vi "3kButtonsSys36x36.vi"() -> ()   [LabVIEW 2011] (continued)
  in  "folder_bell":bool
  in  "folder_add":bool
  in  "folder":bool
  in  "fog":bool
  in  "flower":bool
  in  "flood_it":bool
  in  "flickr":bool
  in  "flex_builder":bool
  in  "flex":bool
  in  "flask_empty":bool
  in  "flask":bool
  in  "flashlight_shine":bool
  in  "flashlight":bool
  in  "flashdisk":bool
  in  "flamingo":bool
  in  "flag_zimbabwe":bool
  in  "flag_zambia":bool
  in  "flag_yemen":bool
  in  "flag_yellow":bool
  in  "flag_wwf":bool
  in  "flag_wto":bool
  in  "flag_wallis_and_futuna":bool
  in  "flag_wales":bool
  in  "flag_virgin_islands":bool
  in  "flag_vietnam":bool
  in  "flag_venezuela":bool
  in  "flag_vatican_city":bool
  in  "flag_vanuatu":bool
  in  "flag_uzbekistan":bool
  in  "flag_usa":bool
  in  "flag_uruquay":bool
  in  "flag_united_nations":bool
  in  "flag_united_arab_emirates":bool
  in  "flag_unesco":bool
  in  "flag_ukraine":bool
  in  "flag_uganda":bool
  in  "flag_tuvalu":bool
  in  "flag_turks_and_caicos_islands":bool
  in  "flag_turkmenistan":bool
  in  "flag_turkey":bool
  in  "flag_tunisia":bool
  in  "flag_trinidad_and_tobago":bool
  in  "flag_tonga":bool
  in  "flag_togo":bool
  in  "flag_tibet":bool
  in  "flag_thailand":bool
  in  "flag_tanzania":bool
  in  "flag_tajikistan":bool
  in  "flag_taiwan":bool
  in  "flag_syria":bool
  in  "flag_switzerland":bool
  in  "flag_sweden":bool
  in  "flag_swaziland":bool
  in  "flag_suriname":bool
  in  "flag_sudan":bool
  in  "flag_sri_lanka":bool
  in  "flag_spain":bool
  in  "flag_south_korea":bool
  in  "flag_south_georgia":bool
  in  "flag_south_africa":bool
  in  "flag_somalia":bool
  in  "flag_solomon_islands":bool
  in  "flag_slovenia":bool
  in  "flag_slovakia":bool
  in  "flag_singapore":bool
  in  "flag_sierra_leone":bool
  in  "flag_seychelles":bool
  in  "flag_serbia_montenegro":bool
  in  "flag_senegal":bool
  in  "flag_scotland":bool
  in  "flag_saudi_arabia":bool
  in  "flag_sao_tome_and_principe":bool
  in  "flag_san_marino":bool
  in  "flag_samoa":bool
  in  "flag_saint_vincent_and_grenadines":bool
  in  "flag_saint_pierre_and_miquelon":bool
  in  "flag_saint_lucia":bool
  in  "flag_saint_kitts_and_nevis":bool
  in  "flag_saint_helena":bool
  in  "flag_rwanda":bool
  in  "flag_russia":bool
  in  "flag_romania":bool
  in  "flag_red_cross":bool
  in  "flag_red":bool
  in  "flag_qatar":bool
  in  "flag_purple":bool
  in  "flag_puerto_rico":bool
  in  "flag_portugal":bool
  in  "flag_poland":bool
  in  "flag_pitcairn_islands":bool
  in  "flag_pink":bool
  in  "flag_philippines":bool
  in  "flag_peru":bool
  in  "flag_paraquay":bool
  in  "flag_papua_new_guinea":bool
  in  "flag_panama":bool
  in  "flag_palau":bool
  in  "flag_pakistan":bool
  in  "flag_orange":bool
  in  "flag_oman":bool
  in  "flag_olympic":bool
  in  "flag_norway":bool
  in  "flag_northern_mariana_islands":bool
  in  "flag_north_korea":bool
  in  "flag_norfolk_islands":bool
  in  "flag_niue":bool
  in  "flag_nigeria":bool
  in  "flag_niger":bool
  in  "flag_nicaragua":bool
  in  "flag_new_zealand":bool
  in  "flag_new":bool
  in  "flag_netherlands_antilles":bool
  in  "flag_netherlands":bool
  in  "flag_nepal":bool
  in  "flag_nauru":bool
  in  "flag_nato":bool
  in  "flag_namibia":bool
  in  "flag_mozambique":bool
  in  "flag_morocco":bool
  in  "flag_montserrat":bool
  in  "flag_mongolia":bool
  in  "flag_monaco":bool
  in  "flag_moldova":bool
  in  "flag_micronesia":bool
  in  "flag_mexico":bool
  in  "flag_mauritius":bool
  in  "flag_mauretania":bool
  in  "flag_martinique":bool
  in  "flag_marshall_islands":bool
  in  "flag_malta":bool
  in  "flag_mali":bool
  in  "flag_maledives":bool
  in  "flag_malaysia":bool
  in  "flag_malawi":bool
  in  "flag_madagascar":bool
  in  "flag_macedonia":bool
  in  "flag_macau":bool
  in  "flag_luxembourg":bool
  in  "flag_lithuania":bool
  in  "flag_liechtenstein":bool
  in  "flag_libya":bool
  in  "flag_liberia":bool
  in  "flag_lesotho":bool
  in  "flag_lebanon":bool
  in  "flag_latvia":bool
  in  "flag_laos":bool
  in  "flag_kyrgyzstan":bool
  in  "flag_kuwait":bool
  in  "flag_kiribati":bool
  in  "flag_kenya":bool
  in  "flag_kazakhstan":bool
  in  "flag_jordan":bool
  in  "flag_jersey":bool
  in  "flag_japan":bool
  in  "flag_jamaica":bool
  in  "flag_italy":bool
  in  "flag_israel":bool
  in  "flag_isle_of_man":bool
  in  "flag_ireland":bool
  in  "flag_iraq":bool
  in  "flag_iran":bool
  in  "flag_indonesia":bool
  in  "flag_india":bool
  in  "flag_iceland":bool
  in  "flag_hungary":bool
  in  "flag_hot":bool
  in  "flag_hong_kong":bool
  in  "flag_honduras":bool
  in  "flag_haiti":bool
  in  "flag_guyana":bool
  in  "flag_guinea_bissau":bool
  in  "flag_guinea":bool
  in  "flag_guernsey":bool
  in  "flag_guatemala":bool
  in  "flag_guam":bool
  in  "flag_grenada":bool
  in  "flag_greenland":bool
  in  "flag_green":bool
  in  "flag_greece":bool
  in  "flag_great_britain":bool
  in  "flag_gibraltar":bool
  in  "flag_ghana":bool
  in  "flag_germany":bool
  in  "flag_georgia":bool
  in  "flag_gambia":bool
  in  "flag_gabon":bool
  in  "flag_french_polynesia":bool
  in  "flag_france":bool
  in  "flag_finland":bool
  in  "flag_finish":bool
  in  "flag_fiji":bool
  in  "flag_faroe_islands":bool
  in  "flag_falkland_islands":bool
  in  "flag_european_union":bool
  in  "flag_ethiopia":bool
  in  "flag_estonia":bool
  in  "flag_eritrea":bool
  in  "flag_equatorial_guinea":bool
  in  "flag_equador":bool
  in  "flag_england":bool
  in  "flag_el_salvador":bool
  in  "flag_egypt":bool
  in  "flag_east_timor":bool
  in  "flag_dominican_republic":bool
  in  "flag_dominica":bool
  in  "flag_djibouti":bool
  in  "flag_denmark":bool
  in  "flag_czech_republic":bool
  in  "flag_cyprus":bool
  in  "flag_cuba":bool
  in  "flag_croatia":bool
  in  "flag_cote_divoire":bool
  in  "flag_costa_rica":bool
  in  "flag_cope_verde":bool
  in  "flag_cook_islands":bool
  in  "flag_congo_republic":bool
  in  "flag_congo_democratic_republic":bool
  in  "flag_comoros":bool
  in  "flag_colombia":bool
  in  "flag_china":bool
  in  "flag_chile":bool
  in  "flag_chad":bool
  in  "flag_central_african_republic":bool
  in  "flag_cayman_islands":bool
  in  "flag_canada":bool
  in  "flag_cameroon":bool
  in  "flag_cambodia":bool
  in  "flag_burundi":bool
  in  "flag_burma":bool
  in  "flag_burkina_faso":bool
  in  "flag_bulgaria":bool
  in  "flag_brunei":bool
  in  "flag_british_virgin_islands":bool
  in  "flag_british_indian_ocean":bool
  in  "flag_brazil":bool
  in  "flag_boy_scout":bool
  in  "flag_botswana":bool
  in  "flag_bosnia":bool
  in  "flag_bolivia":bool
  in  "flag_blue":bool
  in  "flag_bhutan":bool
  in  "flag_bermuda":bool
  in  "flag_benin":bool
  in  "flag_belize":bool
  in  "flag_belgium":bool
  in  "flag_belarus":bool
  in  "flag_barbados":bool
  in  "flag_bangladesh":bool
  in  "flag_bahrain":bool
  in  "flag_bahamas":bool
  in  "flag_azerbaijan":bool
  in  "flag_austria":bool
  in  "flag_australia":bool
  in  "flag_aruba":bool
  in  "flag_armenia":bool
  in  "flag_argentina":bool
  in  "flag_antigua_and_barbuda":bool
  in  "flag_anguilla":bool
  in  "flag_angola":bool
  in  "flag_andorra":bool
  in  "flag_american_samoa":bool
  in  "flag_algeria":bool
  in  "flag_albania":bool
  in  "flag_airfield_vehicle_safety":bool
  in  "flag_afghanistan":bool
  in  "flag_3":bool
  in  "flag_2":bool
  in  "flag_1":bool
  in  "fishfinder":bool
  in  "firewall_burn":bool
  in  "firewall":bool
  in  "firefox":bool
  in  "fire_extinguisher":bool
  in  "fire_damage":bool
  in  "fire":bool
  in  "fingerprint":bool
  in  "find":bool
  in  "finance":bool
  in  "filter_delete":bool
  in  "filter_add":bool
  in  "filter":bool
  in  "film_save":bool
  in  "film_photo":bool
  in  "film_link":bool
  in  "film_key":bool
  in  "film_go":bool
  in  "film_error":bool
  in  "film_edit":bool
  in  "film_delete":bool
  in  "film_add":bool
  in  "film":bool
  in  "fill":bool
  in  "file_manager":bool
  in  "file_extension_zip":bool
  in  "file_extension_xpi":bool
  in  "file_extension_xls":bool
  in  "file_extension_wps":bool
  in  "file_extension_wmv":bool
  in  "file_extension_wma":bool
  in  "file_extension_wav":bool
  in  "file_extension_vob":bool
  in  "file_extension_vcd":bool
  in  "file_extension_txt":bool
  in  "file_extension_ttf":bool
  in  "file_extension_torrent":bool
  in  "file_extension_tmp":bool
  in  "file_extension_tif":bool
  in  "file_extension_thm":bool
  in  "file_extension_tgz":bool
  in  "file_extension_swf":bool
  in  "file_extension_ss":bool
  in  "file_extension_sitx":bool
  in  "file_extension_sit":bool
  in  "file_extension_ses":bool
  in  "file_extension_sea":bool
  in  "file_extension_rtf":bool
  in  "file_extension_rmvb":bool
  in  "file_extension_rm":bool
  in  "file_extension_rar":bool
  in  "file_extension_ram":bool
  in  "file_extension_qxd":bool
  in  "file_extension_qbw":bool
  in  "file_extension_qbb":bool
  in  "file_extension_pub":bool
  in  "file_extension_ptb":bool
  in  "file_extension_pst":bool
  in  "file_extension_psd":bool
  in  "file_extension_ps":bool
  in  "file_extension_pps":bool
  in  "file_extension_png":bool
  in  "file_extension_pdf":bool
  in  "file_extension_ogg":bool
  in  "file_extension_mswmm":bool
  in  "file_extension_msi":bool
  in  "file_extension_mpg":bool
  in  "file_extension_mpeg":bool
  in  "file_extension_mp4":bool
  in  "file_extension_mp2":bool
  in  "file_extension_mov":bool
  in  "file_extension_mid":bool
  in  "file_extension_mdb":bool
  in  "file_extension_mcd":bool
  in  "file_extension_m4v":bool
  in  "file_extension_m4p":bool
  in  "file_extension_m4b":bool
  in  "file_extension_m4a":bool
  in  "file_extension_log":bool
  in  "file_extension_lnk":bool
  in  "file_extension_jpg":bool
  in  "file_extension_jpeg":bool
  in  "file_extension_jar":bool
  in  "file_extension_iso":bool
  in  "file_extension_indd":bool
  in  "file_extension_ifo":bool
  in  "file_extension_html":bool
  in  "file_extension_htm":bool
  in  "file_extension_hqx":bool
  in  "file_extension_gz":bool
  in  "file_extension_gif":bool
  in  "file_extension_flv":bool
  in  "file_extension_fla":bool
  in  "file_extension_exe":bool
  in  "file_extension_eps":bool
  in  "file_extension_eml":bool
  in  "file_extension_dwg":bool
  in  "file_extension_dvf":bool
  in  "file_extension_dss":bool
  in  "file_extension_doc":bool
  in  "file_extension_dmg":bool
  in  "file_extension_dll":bool
  in  "file_extension_divx":bool
  in  "file_extension_dat":bool
  in  "file_extension_chm":bool
  in  "file_extension_cdr":bool
  in  "file_extension_cdl":bool
  in  "file_extension_cda":bool
  in  "file_extension_cbr":bool
  in  "file_extension_cab":bool
  in  "file_extension_bup":bool
  in  "file_extension_bmp":bool
  in  "file_extension_bin":bool
  in  "file_extension_bat":bool
  in  "file_extension_asx":bool
  in  "file_extension_asf":bool
  in  "file_extension_amr":bool
  in  "file_extension_aiff":bool
  in  "file_extension_aif":bool
  in  "file_extension_ai":bool
  in  "file_extension_ace":bool
  in  "file_extension_7z":bool
  in  "file_extension_3gp":bool
  in  "female":bool
  in  "feed_magnify":bool
  in  "feed_key":bool
  in  "feed_go":bool
  in  "feed_error":bool
  in  "feed_edit":bool
  in  "feed_disk":bool
  in  "feed_delete":bool
  in  "feed_add":bool
  in  "feed":bool
  in  "fedora":bool
  in  "fax":bool
  in  "fatcow":bool
  in  "factory":bool
  in  "facebook":bool
  in  "faberge_egg":bool
  in  "eye_red":bool
  in  "eye_close":bool
  in  "eye":bool
  in  "extract_foreground_objects":bool
  in  "external":bool
  in  "export_excel":bool
  in  "exclamation":bool
  in  "evernote":bool
  in  "events":bool
  in  "evacuator":bool
  in  "escimo_pie":bool
  in  "error_go":bool
  in  "error_delete":bool
  in  "error_add":bool
  in  "error":bool
  in  "envelope_string":bool
  in  "envelope":bool
  in  "entity":bool
  in  "emotion_zedz":bool
  in  "emotion_wink":bool
  in  "emotion_whist":bool
  in  "emotion_what":bool
  in  "emotion_waii":bool
  in  "emotion_waaaht":bool
  in  "emotion_vampire":bool
  in  "emotion_unshaven":bool
  in  "emotion_unhappy":bool
  in  "emotion_too_sad":bool
  in  "emotion_tongue":bool
  in  "emotion_tire":bool
  in  "emotion_terminator":bool
  in  "emotion_sweat":bool
  in  "emotion_surrender":bool
  in  "emotion_sure":bool
  in  "emotion_suprised":bool
  in  "emotion_stupid":bool
  in  "emotion_star":bool
  in  "emotion_spy":bool
  in  "emotion_spiderman":bool
  in  "emotion_smile":bool
  in  "emotion_sleep":bool
  in  "emotion_skull":bool
  in  "emotion_silent":bool
  in  "emotion_sick":bool
  in  "emotion_shocked":bool
  in  "emotion_shame":bool
  in  "emotion_sad":bool
  in  "emotion_red":bool
  in  "emotion_rap":bool
  in  "emotion_question":bool
  in  "emotion_pumpkin":bool
  in  "emotion_pirate":bool
  in  "emotion_nosebleed":bool
  in  "emotion_ninja":bool
  in  "emotion_nerd":bool
  in  "emotion_mummy":bool
  in  "emotion_money":bool
  in  "emotion_misdoubt":bool
  in  "emotion_medic":bool
  in  "emotion_matrix":bool
  in  "emotion_mad":bool
  in  "emotion_love":bool
  in  "emotion_kissed":bool
  in  "emotion_kiss":bool
  in  "emotion_jason":bool
  in  "emotion_japan":bool
  in  "emotion_hypnotized":bool
  in  "emotion_hungry":bool
  in  "emotion_horror":bool
  in  "emotion_hitler":bool
  in  "emotion_happy":bool
  in  "emotion_hand_flower":bool
  in  "emotion_haha":bool
  in  "emotion_grin":bool
  in  "emotion_greedy":bool
  in  "emotion_go":bool
  in  "emotion_girl":bool
  in  "emotion_ghost":bool
  in  "emotion_gear":bool
  in  "emotion_franken":bool
  in  "emotion_flower_dead":bool
  in  "emotion_fan":bool
  in  "emotion_face_panda":bool
  in  "emotion_face_monkey":bool
  in  "emotion_eyes_droped":bool
  in  "emotion_exciting":bool
  in  "emotion_evolution":bool
  in  "emotion_evilgrin":bool
  in  "emotion_dribble":bool
  in  "emotion_doubt":bool
  in  "emotion_diver":bool
  in  "emotion_devil":bool
  in  "emotion_dead":bool
  in  "emotion_david_blaine":bool
  in  "emotion_darth_wader":bool
  in  "emotion_cyclops":bool
  in  "emotion_cry":bool
  in  "emotion_crazy_rabbit":bool
  in  "emotion_crazy":bool
  in  "emotion_cool":bool
  in  "emotion_confuse":bool
  in  "emotion_confident":bool
  in  "emotion_cold":bool
  in  "emotion_clown":bool
  in  "emotion_bye_bye":bool
  in  "emotion_bubblegum":bool
  in  "emotion_bloody":bool
  in  "emotion_bigsmile":bool
  in  "emotion_beaten":bool
  in  "emotion_beat_brick":bool
  in  "emotion_batman":bool
  in  "emotion_baffle":bool
  in  "emotion_bad_smelly":bool
  in  "emotion_bad_egg":bool
  in  "emotion_baby":bool
  in  "emotion_angry":bool
  in  "emotion_anger":bool
  in  "emotion_angel":bool
  in  "emotion_amazing":bool
  in  "emotion_alien":bool
  in  "emotion_ah":bool
  in  "emotion_after_boom":bool
  in  "emotion_adore":bool
  in  "ember":bool
  in  "emails_stack":bool
  in  "emails":bool
  in  "email_to_friend":bool
  in  "email_send_receive":bool
  in  "email_open_image":bool
  in  "email_open":bool
  in  "email_link":bool
  in  "email_go":bool
  in  "email_forward":bool
  in  "email_error":bool
  in  "email_edit":bool
  in  "email_delete":bool
  in  "email_attach":bool
  in  "email_at_sign":bool
  in  "email_air":bool
  in  "email_add":bool
  in  "email":bool
  in  "elements":bool
  in  "electric_guitar":bool
  in  "ehow":bool
  in  "egyptian_pyramid":bool
  in  "education":bool
  in  "edit_path":bool
  in  "edit_mathematics":bool
  in  "edit_free":bool
  in  "edit_diff":bool
  in  "edit_chain":bool
  in  "echeck":bool
  in  "ebay":bool
  in  "earth_night":bool
  in  "ear_listen":bool
  in  "e_book_reader_white":bool
  in  "e_book_reader_black":bool
  in  "dynamite":bool
  in  "dvd_link":bool
  in  "dvd_key":bool
  in  "dvd_go":bool
  in  "dvd_error":bool
  in  "dvd_edit":bool
  in  "dvd_delete":bool
  in  "dvd_add":bool
  in  "dvd":bool
  in  "drum":bool
  in  "drugs_com":bool
  in  "drop":bool
  in  "drive_web":bool
  in  "drive_user":bool
  in  "drive_rename":bool
  in  "drive_network":bool
  in  "drive_magnify":bool
  in  "drive_link":bool
  in  "drive_key":bool
  in  "drive_go":bool
  in  "drive_error":bool
  in  "drive_edit":bool
  in  "drive_disk":bool
  in  "drive_delete":bool
  in  "drive_cd_empty":bool
  in  "drive_cd":bool
  in  "drive_burn":bool
  in  "drive_add":bool
  in  "drive":bool
  in  "drink_empty":bool
  in  "drink":bool
  in  "drill":bool
  in  "dribbble":bool
  in  "drawer_open":bool
  in  "drawer":bool
  in  "draw_wave":bool
  in  "draw_vertex":bool
  in  "draw_star":bool
  in  "draw_spiral":bool
  in  "draw_smudge":bool
  in  "draw_ring":bool
  in  "draw_polyline":bool
  in  "draw_polygon_curves":bool
  in  "draw_polygon":bool
  in  "draw_points":bool
  in  "draw_path":bool
  in  "draw_line":bool
  in  "draw_island":bool
  in  "draw_ink":bool
  in  "draw_eraser":bool
  in  "draw_ellipse":bool
  in  "draw_dodge_burn":bool
  in  "draw_convolve":bool
  in  "draw_clone":bool
  in  "draw_calligraphic":bool
  in  "draw_airbrush":bool
  in  "download_for_windows":bool
  in  "download_for_mac":bool
  in  "download_for_linux":bool
  in  "download_cloud":bool
  in  "download":bool
  in  "down_jacket":bool
  in  "dopplr":bool
  in  "door_out":bool
  in  "door_open":bool
  in  "door_in":bool
  in  "door":bool
  in  "donut":bool
  in  "domain_template":bool
  in  "domain_names_advanced":bool
  in  "domain_name_monetization":bool
  in  "domain_name_investment":bool
  in  "domain_legal_issues":bool
  in  "domain_controversies":bool
  in  "domain_buying_selling":bool
  in  "dog":bool
  in  "documents_email":bool
  in  "document_yellow":bool
  in  "document_white_torn":bool
  in  "document_view_book":bool
  in  "document_vertical":bool
  in  "document_valid":bool
  in  "document_tree":bool
  in  "document_torn":bool
  in  "document_todo":bool
  in  "document_tag":bool
  in  "document_stand":bool
  in  "document_split":bool
  in  "document_spacing":bool
  in  "document_signature":bool
  in  "document_shred":bool
  in  "document_shapes":bool
  in  "document_rename":bool
  in  "document_redirect":bool
  in  "document_red":bool
  in  "document_quote":bool
  in  "document_properties":bool
  in  "document_prepare":bool
  in  "document_plus":bool
  in  "document_page_previous":bool
  in  "document_page_next":bool
  in  "document_page_last":bool
  in  "document_page":bool
  in  "document_num":bool
  in  "document_notes":bool
  in  "document_next":bool
  in  "document_move":bool
  in  "document_mark_as_final":bool
  in  "document_margins":bool
  in  "document_layout":bool
  in  "document_inspector":bool
  in  "document_inspect":bool
  in  "document_insert":bool
  in  "document_info":bool
  in  "document_index":bool
  in  "document_import":bool
  in  "document_image_ver":bool
  in  "document_image_hor":bool
  in  "document_image":bool
  in  "document_green":bool
  in  "document_font_wizard":bool
  in  "document_font":bool
  in  "document_export":bool
  in  "document_empty":bool
  in  "document_editing":bool
  in  "document_copies":bool
  in  "document_comments":bool
  in  "document_comment_below":bool
  in  "document_comment_behind":bool
  in  "document_comment_above":bool
  in  "document_check_compatibility":bool
  in  "document_center":bool
  in  "document_break":bool
  in  "document_black":bool
  in  "document_background":bool
  in  "document_back":bool
  in  "do_not_disturb":bool
  in  "dns_setting":bool
  in  "dns":bool
  in  "distribution_partnerships":bool
  in  "disk_multiple":bool
  in  "disk":bool
  in  "dish":bool
  in  "discover":bool
  in  "disconnect":bool
  in  "directory_listing":bool
  in  "direction":bool
  in  "dinersclub":bool
  in  "digital_signature_pen":bool
  in  "digital_signature":bool
  in  "digg":bool
  in  "dice":bool
  in  "diamond":bool
  in  "dialog":bool
  in  "diagramm":bool
  in  "diagnostic_chart":bool
  in  "devianart":bool
  in  "desktop":bool
  in  "designmoo":bool
  in  "design_float":bool
  in  "derivatives":bool
  in  "delicious":bool
  in  "delete":bool
  in  "decimal_more":bool
  in  "decimal_less":bool
  in  "debian":bool
  in  "ddr_memory":bool
  in  "date_task":bool
  in  "date_relation":bool
  in  "date_previous_gray":bool
  in  "date_previous":bool
  in  "date_next_gray":bool
  in  "date_next":bool
  in  "date_magnify":bool
  in  "date_link":bool
  in  "date_go":bool
  in  "date_error":bool
  in  "date_edit":bool
  in  "date_delete":bool
  in  "date_add":bool
  in  "date":bool
  in  "database_yellow":bool
  in  "database_table":bool
  in  "database_server":bool
  in  "database_save":bool
  in  "database_refresh":bool
  in  "database_red":bool
  in  "database_link":bool
  in  "database_lightning":bool
  in  "database_key":bool
  in  "database_green":bool
  in  "database_go":bool
  in  "database_gear":bool
  in  "database_error":bool
  in  "database_edit":bool
  in  "database_delete":bool
  in  "database_connect":bool
  in  "database_blue":bool
  in  "database_black":bool
  in  "database_add":bool
  in  "database":bool
  in  "data_table":bool
  in  "data_sort":bool
  in  "data_grid":bool
  in  "data_field":bool
  in  "data_chooser":bool
  in  "dashboard":bool
  in  "cutter":bool
  in  "cutlery":bool
  in  "cutleries":bool
  in  "cut_red":bool
  in  "cut":bool
  in  "cushion":bool
  in  "curtain":bool
  in  "cursor":bool
  in  "curriculum_vitae":bool
  in  "cup_silver":bool
  in  "cup_link":bool
  in  "cup_key":bool
  in  "cup_gold":bool
  in  "cup_go":bool
  in  "cup_error":bool
  in  "cup_edit":bool
  in  "cup_delete":bool
  in  "cup_bronze":bool
  in  "cup_add":bool
  in  "cup":bool
  in  "css_valid":bool
  in  "css_go":bool
  in  "css_delete":bool
  in  "css_add":bool
  in  "css_3":bool
  in  "css":bool
  in  "cruise_ship":bool
  in  "crown_silver":bool
  in  "crown_gold":bool
  in  "crown_bronze":bool
  in  "cross_shield":bool
  in  "cross_promotion_selling":bool
  in  "cross":bool
  in  "cricket":bool
  in  "creditcards":bool
  in  "credit":bool
  in  "creative_commons":bool
  in  "counter":bool
  in  "copyleft":bool
  in  "copying_and_distribution":bool
  in  "cooler":bool
  in  "cookies":bool
  in  "cookie_chocolate":bool
  in  "convert_gray_to_color":bool
  in  "convert_color_to_gray":bool
  in  "conversion_of_currency":bool
  in  "controller_error":bool
  in  "controller_delete":bool
  in  "controller_add":bool
  in  "controller":bool
  in  "controlbar":bool
  in  "control_stop_blue":bool
  in  "control_stop":bool
  in  "control_start_blue":bool
  in  "control_start":bool
  in  "control_rewind_blue":bool
  in  "control_rewind":bool
  in  "control_repeat_blue":bool
  in  "control_repeat":bool
  in  "control_power_blue":bool
  in  "control_power":bool
  in  "control_play_blue":bool
  in  "control_play":bool
  in  "control_pause_record":bool
  in  "control_pause_blue":bool
  in  "control_pause":bool
  in  "control_panel_branding":bool
  in  "control_panel_access":bool
  in  "control_panel":bool
  in  "control_fastforward_blue":bool
  in  "control_fastforward":bool
  in  "control_equalizer_blue":bool
  in  "control_equalizer":bool
  in  "control_end_blue":bool
  in  "control_end":bool
  in  "control_eject_blue":bool
  in  "control_eject":bool
  in  "control_cursor_blue":bool
  in  "control_cursor":bool
  in  "contrast_low":bool
  in  "contrast_increase":bool
  in  "contrast_high":bool
  in  "contrast_decrease":bool
  in  "contrast":bool
  in  "contact_email":bool
  in  "construction":bool
  in  "connect":bool
  in  "computer_link":bool
  in  "computer_key":bool
  in  "computer_go":bool
  in  "computer_error":bool
  in  "computer_edit":bool
  in  "computer_delete":bool
  in  "computer_add":bool
  in  "computer":bool
  in  "compress":bool
  in  "compile_warning":bool
  in  "compile_error":bool
  in  "compile":bool
  in  "compass":bool
  in  "company_generosity":bool
  in  "comments_twitter":bool
  in  "comments_facebook":bool
  in  "comments_delete":bool
  in  "comments_add":bool
  in  "comments":bool
  in  "comment_white":bool
  in  "comment_twitter_retwit":bool
  in  "comment_twitter_box":bool
  in  "comment_twitter":bool
  in  "comment_google":bool
  in  "comment_facebook_box":bool
  in  "comment_facebook":bool
  in  "comment_edit":bool
  in  "comment_delete":bool
  in  "comment_box":bool
  in  "comment_add":bool
  in  "comment":bool
  in  "combo_box":bool
  in  "columnchart":bool
  in  "column_two":bool
  in  "column_tree":bool
  in  "column_single":bool
  in  "column_right":bool
  in  "column_one":bool
  in  "column_left":bool
  in  "column_four":bool
  in  "column_double":bool
  in  "color_wheel":bool
  in  "color_swatches":bool
  in  "color_swatch":bool
  in  "color_picker_alternative":bool
  in  "color_picker":bool
  in  "color_management":bool
  in  "color_gradient":bool
  in  "color_adjustment_red":bool
  in  "color_adjustment_green":bool
  in  "color_adjustment_blue":bool
  in  "color_adjustment":bool
  in  "cold":bool
  in  "coins_in_hand":bool
  in  "coins_delete":bool
  in  "coins_add":bool
  in  "coins":bool
  in  "coin_stack_gold":bool
  in  "coin_single_silver":bool
  in  "coin_single_gold":bool
  in  "coin_single_cooper":bool
  in  "cog_go":bool
  in  "cog_error":bool
  in  "cog_edit":bool
  in  "cog_delete":bool
  in  "cog_add":bool
  in  "cog":bool
  in  "code":bool
  in  "cocacola":bool
  in  "co2":bool
  in  "clown_fish":bool
  in  "clock_stop":bool
  in  "clock_select_remain":bool
  in  "clock_red":bool
  in  "clock_play":bool
  in  "clock_pause":bool
  in  "clock_moon_phase":bool
  in  "clock_link":bool
  in  "clock_history_frame":bool
  in  "clock_go":bool
  in  "clock_error":bool
  in  "clock_edit":bool
  in  "clock_delete":bool
  in  "clock_add":bool
  in  "clock_45":bool
  in  "clock_15":bool
  in  "clock_":bool
  in  "clipboard_sign_out":bool
  in  "clipboard_sign":bool
  in  "clipboard_invoice":bool
  in  "clipboard_empty":bool
  in  "clip_splitter":bool
  in  "client_account_template":bool
  in  "cirrus":bool
  in  "circus":bool
  in  "cinema_ticket":bool
  in  "cigarette":bool
  in  "church":bool
  in  "christmas_tree":bool
  in  "chocolate_bite":bool
  in  "chocolate":bool
  in  "chinese_noodles":bool
  in  "children_cap":bool
  in  "chiken_leg":bool
  in  "chess_tower":bool
  in  "chess_horse":bool
  in  "cheque":bool
  in  "chefs_hat":bool
  in  "cheese":bool
  in  "checkerboard":bool
  in  "check_box":bool
  in  "chartplotter":bool
  in  "chart_up_color":bool
  in  "chart_stock":bool
  in  "chart_pie_link":bool
  in  "chart_pie_error":bool
  in  "chart_pie_edit":bool
  in  "chart_pie_delete":bool
  in  "chart_pie_alternative":bool
  in  "chart_pie_add":bool
  in  "chart_pie":bool
  in  "chart_organisation_delete":bool
  in  "chart_organisation_add":bool
  in  "chart_organisation":bool
  in  "chart_line_link":bool
  in  "chart_line_error":bool
  in  "chart_line_edit":bool
  in  "chart_line_delete":bool
  in  "chart_line_add":bool
  in  "chart_line":bool
  in  "chart_down_color":bool
  in  "chart_curve_link":bool
  in  "chart_curve_go":bool
  in  "chart_curve_error":bool
  in  "chart_curve_edit":bool
  in  "chart_curve_delete":bool
  in  "chart_curve_add":bool
  in  "chart_curve":bool
  in  "chart_column_2":bool
  in  "chart_column":bool
  in  "chart_bullseye":bool
  in  "chart_bar_link":bool
  in  "chart_bar_error":bool
  in  "chart_bar_edit":bool
  in  "chart_bar_delete":bool
  in  "chart_bar_add":bool
  in  "chart_bar":bool
  in  "change_password":bool
  in  "chameleon":bool
  in  "chair":bool
  in  "ceo":bool
  in  "centroid":bool
  in  "centos":bool
  in  "celsius":bool
  in  "cd_go":bool
  in  "cd_eject":bool
  in  "cd_edit":bool
  in  "cd_delete":bool
  in  "cd_case_empty":bool
  in  "cd_case":bool
  in  "cd_burn":bool
  in  "cd_add":bool
  in  "cd":bool
  in  "cctv_camera":bool
  in  "caution_radiation":bool
  in  "caution_high_voltage":bool
  in  "caution_board":bool
  in  "caution_biohazard":bool
  in  "cats_display":bool
  in  "caterpillar":bool
  in  "category_item_select":bool
  in  "category_item":bool
  in  "category_group_select":bool
  in  "category_group":bool
  in  "category":bool
  in  "categories":bool
  in  "cat":bool
  in  "cash_terminal":bool
  in  "cash_stack":bool
  in  "cash_register_2":bool
  in  "cash_register":bool
  in  "cart_remove":bool
  in  "cart_put":bool
  in  "cart_go":bool
  in  "cart_full":bool
  in  "cart_error":bool
  in  "cart_edit":bool
  in  "cart_delete":bool
  in  "cart_add":bool
  in  "cart":bool
  in  "cargo":bool
  in  "cards_binds":bool
  in  "cards_bind_address":bool
  in  "cards":bool
  in  "card_solo":bool
  in  "card_save":bool
  in  "card_sapphire":bool
  in  "card_money":bool
  in  "card_miles":bool
  in  "card_ipod":bool
  in  "card_import":bool
  in  "card_gold":bool
  in  "card_gift_2":bool
  in  "card_gift":bool
  in  "card_front":bool
  in  "card_export":bool
  in  "card_echeck":bool
  in  "card_discover_novus":bool
  in  "card_discover_black":bool
  in  "card_debit":bool
  in  "card_credit":bool
  in  "card_chip_silver":bool
  in  "card_chip_gold":bool
  in  "card_chase":bool
  in  "card_bank":bool
  in  "card_back":bool
  in  "card_apple":bool
  in  "card_amex_green":bool
  in  "card_amex_gray":bool
  in  "card_amex_gold":bool
  in  "card_amazon":bool
  in  "car_taxi":bool
  in  "car_delete":bool
  in  "car_add":bool
  in  "car":bool
  in  "cap":bool
  in  "canvas_size":bool
  in  "canvas":bool
  in  "candy_cane":bool
  in  "candlestickchart":bool
  in  "candle_2":bool
  in  "candle":bool
  in  "cancel":bool
  in  "camera_small":bool
  in  "camera_link":bool
  in  "camera_lens":bool
  in  "camera_go":bool
  in  "camera_error":bool
  in  "camera_edit":bool
  in  "camera_delete":bool
  in  "camera_black":bool
  in  "camera_add":bool
  in  "camera":bool
  in  "camcorder":bool
  in  "calendar_view_week":bool
  in  "calendar_view_month":bool
  in  "calendar_view_day":bool
  in  "calendar_link":bool
  in  "calendar_edit":bool
  in  "calendar_delete":bool
  in  "calendar_copy":bool
  in  "calendar_add":bool
  in  "calendar":bool
  in  "calculator_link":bool
  in  "calculator_error":bool
  in  "calculator_edit":bool
  in  "calculator_delete":bool
  in  "calculator_black":bool
  in  "calculator_add":bool
  in  "calculator":bool
  in  "cake":bool
  in  "cactus":bool
  in  "buzz":bool
  in  "buttonbar":bool
  in  "button":bool
  in  "butterfly":bool
  in  "bus":bool
  in  "burro":bool
  in  "bullet_yellow":bool
  in  "bullet_wrench":bool
  in  "bullet_world":bool
  in  "bullet_word":bool
  in  "bullet_white":bool
  in  "bullet_vector":bool
  in  "bullet_valid":bool
  in  "bullet_user":bool
  in  "bullet_up":bool
  in  "bullet_toggle_plus":bool
  in  "bullet_toggle_minus":bool
  in  "bullet_textfield":bool
  in  "bullet_table":bool
  in  "bullet_star":bool
  in  "bullet_red":bool
  in  "bullet_purple":bool
  in  "bullet_powerpoint":bool
  in  "bullet_pink":bool
  in  "bullet_picture":bool
  in  "bullet_php":bool
  in  "bullet_palette":bool
  in  "bullet_orange":bool
  in  "bullet_office":bool
  in  "bullet_medal":bool
  in  "bullet_magnify":bool
  in  "bullet_link":bool
  in  "bullet_lightning":bool
  in  "bullet_key":bool
  in  "bullet_green":bool
  in  "bullet_go":bool
  in  "bullet_gear":bool
  in  "bullet_flash":bool
  in  "bullet_find":bool
  in  "bullet_feed":bool
  in  "bullet_excel":bool
  in  "bullet_error":bool
  in  "bullet_edit":bool
  in  "bullet_dvd":bool
  in  "bullet_down":bool
  in  "bullet_document":bool
  in  "bullet_disk":bool
  in  "bullet_delete":bool
  in  "bullet_database":bool
  in  "bullet_connect":bool
  in  "bullet_code_red":bool
  in  "bullet_code":bool
  in  "bullet_chart":bool
  in  "bullet_cd":bool
  in  "bullet_camera":bool
  in  "bullet_burn":bool
  in  "bullet_bulb_on":bool
  in  "bullet_bulb_off":bool
  in  "bullet_bug":bool
  in  "bullet_brush":bool
  in  "bullet_blue":bool
  in  "bullet_black":bool
  in  "bullet_bell":bool
  in  "bullet_back":bool
  in  "bullet_attach":bool
  in  "bullet_arrow_up":bool
  in  "bullet_arrow_top":bool
  in  "bullet_arrow_right_2":bool
  in  "bullet_arrow_right":bool
  in  "bullet_arrow_left_2":bool
  in  "bullet_arrow_left":bool
  in  "bullet_arrow_down":bool
  in  "bullet_arrow_bottom":bool
  in  "bullet_archive":bool
  in  "bullet_add":bool
  in  "bulb":bool
  in  "building_link":bool
  in  "building_key":bool
  in  "building_go":bool
  in  "building_error":bool
  in  "building_edit":bool
  in  "building_delete":bool
  in  "building_add":bool
  in  "building":bool
  in  "bug_link":bool
  in  "bug_go":bool
  in  "bug_error":bool
  in  "bug_edit":bool
  in  "bug_delete":bool
  in  "bug_add":bool
  in  "bug":bool
  in  "bucket_truck":bool
  in  "bubblechart":bool
  in  "brushes":bool
  in  "broom":bool
  in  "brightkite":bool
  in  "briefcase":bool
  in  "bricks":bool
  in  "brick_link":bool
  in  "brick_go":bool
  in  "brick_error":bool
  in  "brick_edit":bool
  in  "brick_delete":bool
  in  "brick_add":bool
  in  "brick":bool
  in  "breeze":bool
  in  "bread":bool
  in  "brain_trainer":bool
  in  "brain":bool
  in  "boxing_glove":bool
  in  "box_search":bool
  in  "box_open":bool
  in  "box_front":bool
  in  "box_down":bool
  in  "box_closed":bool
  in  "box":bool
  in  "bow":bool
  in  "border_color":bool
  in  "border_2_top":bool
  in  "border_2_right":bool
  in  "border_2_outer":bool
  in  "border_2_left":bool
  in  "border_2_bottom":bool
  in  "border_1d_top":bool
  in  "border_1d_right":bool
  in  "border_1d_left":bool
  in  "border_1d_bottom":bool
  in  "border_1d_around":bool
  in  "border_1_ver":bool
  in  "border_1_top":bool
  in  "border_1_right":bool
  in  "border_1_outer":bool
  in  "border_1_none":bool
  in  "border_1_middle":bool
  in  "border_1_left":bool
  in  "border_1_hor":bool
  in  "border_1_bottom":bool
  in  "border_1":bool
  in  "boomerang":bool
  in  "bookshelf":bool
  in  "books_stack":bool
  in  "books":bool
  in  "bookmark_red":bool
  in  "bookmark":bool
  in  "book_spelling":bool
  in  "book_previous":bool
  in  "book_picture":bool
  in  "book_open":bool
  in  "book_next":bool
  in  "book_link":bool
  in  "book_key":bool
  in  "book_keeping":bool
  in  "book_go":bool
  in  "book_error":bool
  in  "book_edit":bool
  in  "book_delete":bool
  in  "book_addresses":bool
  in  "book_add":bool
  in  "book":bool
  in  "bomb":bool
  in  "board_game":bool
  in  "bluetooth":bool
  in  "blueprints":bool
  in  "blueprint_horizontal":bool
  in  "blueprint":bool
  in  "blogs":bool
  in  "blogger":bool
  in  "blackboard_sum":bool
  in  "blackboard_steps":bool
  in  "blackboard_empty":bool
  in  "blackboard_drawing":bool
  in  "blackberry_white":bool
  in  "blackberry_messenger":bool
  in  "blackberry":bool
  in  "bios":bool
  in  "bin_recycle":bool
  in  "bin_empty":bool
  in  "bin_closed":bool
  in  "bin":bool
  in  "billiard_marker":bool
  in  "bell_link":bool
  in  "bell_go":bool
  in  "bell_error":bool
  in  "bell_delete":bool
  in  "bell_add":bool
  in  "bell":bool
  in  "beer":bool
  in  "bedo":bool
  in  "bed":bool
  in  "bean":bool
  in  "beaker_empty":bool
  in  "beaker":bool
  in  "battery_plug":bool
  in  "battery_low":bool
  in  "battery_half":bool
  in  "battery_full":bool
  in  "battery_charge":bool
  in  "battery":bool
  in  "baton":bool
  in  "basket_remove":bool
  in  "basket_put":bool
  in  "basket_go":bool
  in  "basket_full":bool
  in  "basket_error":bool
  in  "basket_edit":bool
  in  "basket_delete":bool
  in  "basket_add":bool
  in  "basket":bool
  in  "barcode_2d":bool
  in  "barcode":bool
  in  "barchart":bool
  in  "bank":bool
  in  "bandaid":bool
  in  "bamboos":bool
  in  "bamboo":bool
  in  "baloon_2_empty":bool
  in  "baloon_2":bool
  in  "baloon":bool
  in  "ballon":bool
  in  "balance_unbalance":bool
  in  "balance":bool
  in  "baggage_cart_box":bool
  in  "baggage_cart":bool
  in  "backup_manager":bool
  in  "backpack":bool
  in  "baby_bottle":bool
  in  "ax":bool
  in  "award_star_silver_3":bool
  in  "award_star_silver_2":bool
  in  "award_star_silver_1":bool
  in  "award_star_gold_3":bool
  in  "award_star_gold_2":bool
  in  "award_star_gold_1":bool
  in  "award_star_delete":bool
  in  "award_star_bronze_3":bool
  in  "award_star_bronze_2":bool
  in  "award_star_bronze_1":bool
  in  "award_star_add":bool
  in  "autos":bool
  in  "auction_hammer_gavel":bool
  in  "attribution":bool
  in  "attributes_display":bool
  in  "attach":bool
  in  "atm":bool
  in  "at_sign":bool
  in  "asterisk_yellow":bool
  in  "asterisk_orange":bool
  in  "ask_and_answer":bool
  in  "artwork":bool
  in  "arrow_up":bool
  in  "arrow_undo":bool
  in  "arrow_turn_right":bool
  in  "arrow_turn_left":bool
  in  "arrow_switch":bool
  in  "arrow_rotate_clockwise":bool
  in  "arrow_rotate_anticlockwise":bool
  in  "arrow_right":bool
  in  "arrow_refresh_small":bool
  in  "arrow_refresh":bool
  in  "arrow_redo":bool
  in  "arrow_out":bool
  in  "arrow_merge":bool
  in  "arrow_left":bool
  in  "arrow_join":bool
  in  "arrow_inout":bool
  in  "arrow_in":bool
  in  "arrow_down":bool
  in  "arrow_divide":bool
  in  "arrow_branch":bool
  in  "areachart":bool
  in  "arch_linux":bool
  in  "application_xp_terminal":bool
  in  "application_xp":bool
  in  "application_view_tile":bool
  in  "application_view_list":bool
  in  "application_view_icons":bool
  in  "application_view_gallery":bool
  in  "application_view_detail":bool
  in  "application_view_columns":bool
  in  "application_tile_vertical":bool
  in  "application_tile_horizontal":bool
  in  "application_split":bool
  in  "application_side_tree":bool
  in  "application_side_list":bool
  in  "application_side_expand":bool
  in  "application_side_contract":bool
  in  "application_side_boxes":bool
  in  "application_put":bool
  in  "application_osx_terminal":bool
  in  "application_osx":bool
  in  "application_link":bool
  in  "application_lightning":bool
  in  "application_key":bool
  in  "application_home":bool
  in  "application_go":bool
  in  "application_get":bool
  in  "application_from_storage":bool
  in  "application_form_magnify":bool
  in  "application_form_edit":bool
  in  "application_form_delete":bool
  in  "application_form_add":bool
  in  "application_form":bool
  in  "application_error":bool
  in  "application_edit":bool
  in  "application_double":bool
  in  "application_delete":bool
  in  "application_control_bar":bool
  in  "application_cascade":bool
  in  "application_add":bool
  in  "application":bool
  in  "apple_half":bool
  in  "apple_corp":bool
  in  "apple":bool
  in  "aol_messenger":bool
  in  "aol_mail":bool
  in  "anti_xss":bool
  in  "angel":bool
  in  "android":bool
  in  "anchor":bool
  in  "american_express":bool
  in  "all_right_reserved":bool
  in  "alitalk":bool
  in  "align_right":bool
  in  "align_none":bool
  in  "align_middle":bool
  in  "align_left":bool
  in  "align_compact":bool
  in  "align_center":bool
  in  "align_bellow":bool
  in  "align_above":bool
  in  "alarm_bell":bool
  in  "aim_messenger":bool
  in  "agp":bool
  in  "advertising":bool
  in  "advanced_data_grid":bool
  in  "administrator":bool
  in  "add":bool
  in  "active_sessions":bool
  in  "action_log":bool
  in  "acoustic_guitar":bool
  in  "acorn":bool
  in  "account_balances":bool
  in  "accordion":bool
  in  "accept":bool
  in  "64_bit":bool
  in  "32_bit":bool
  in  "3d_glasses":bool
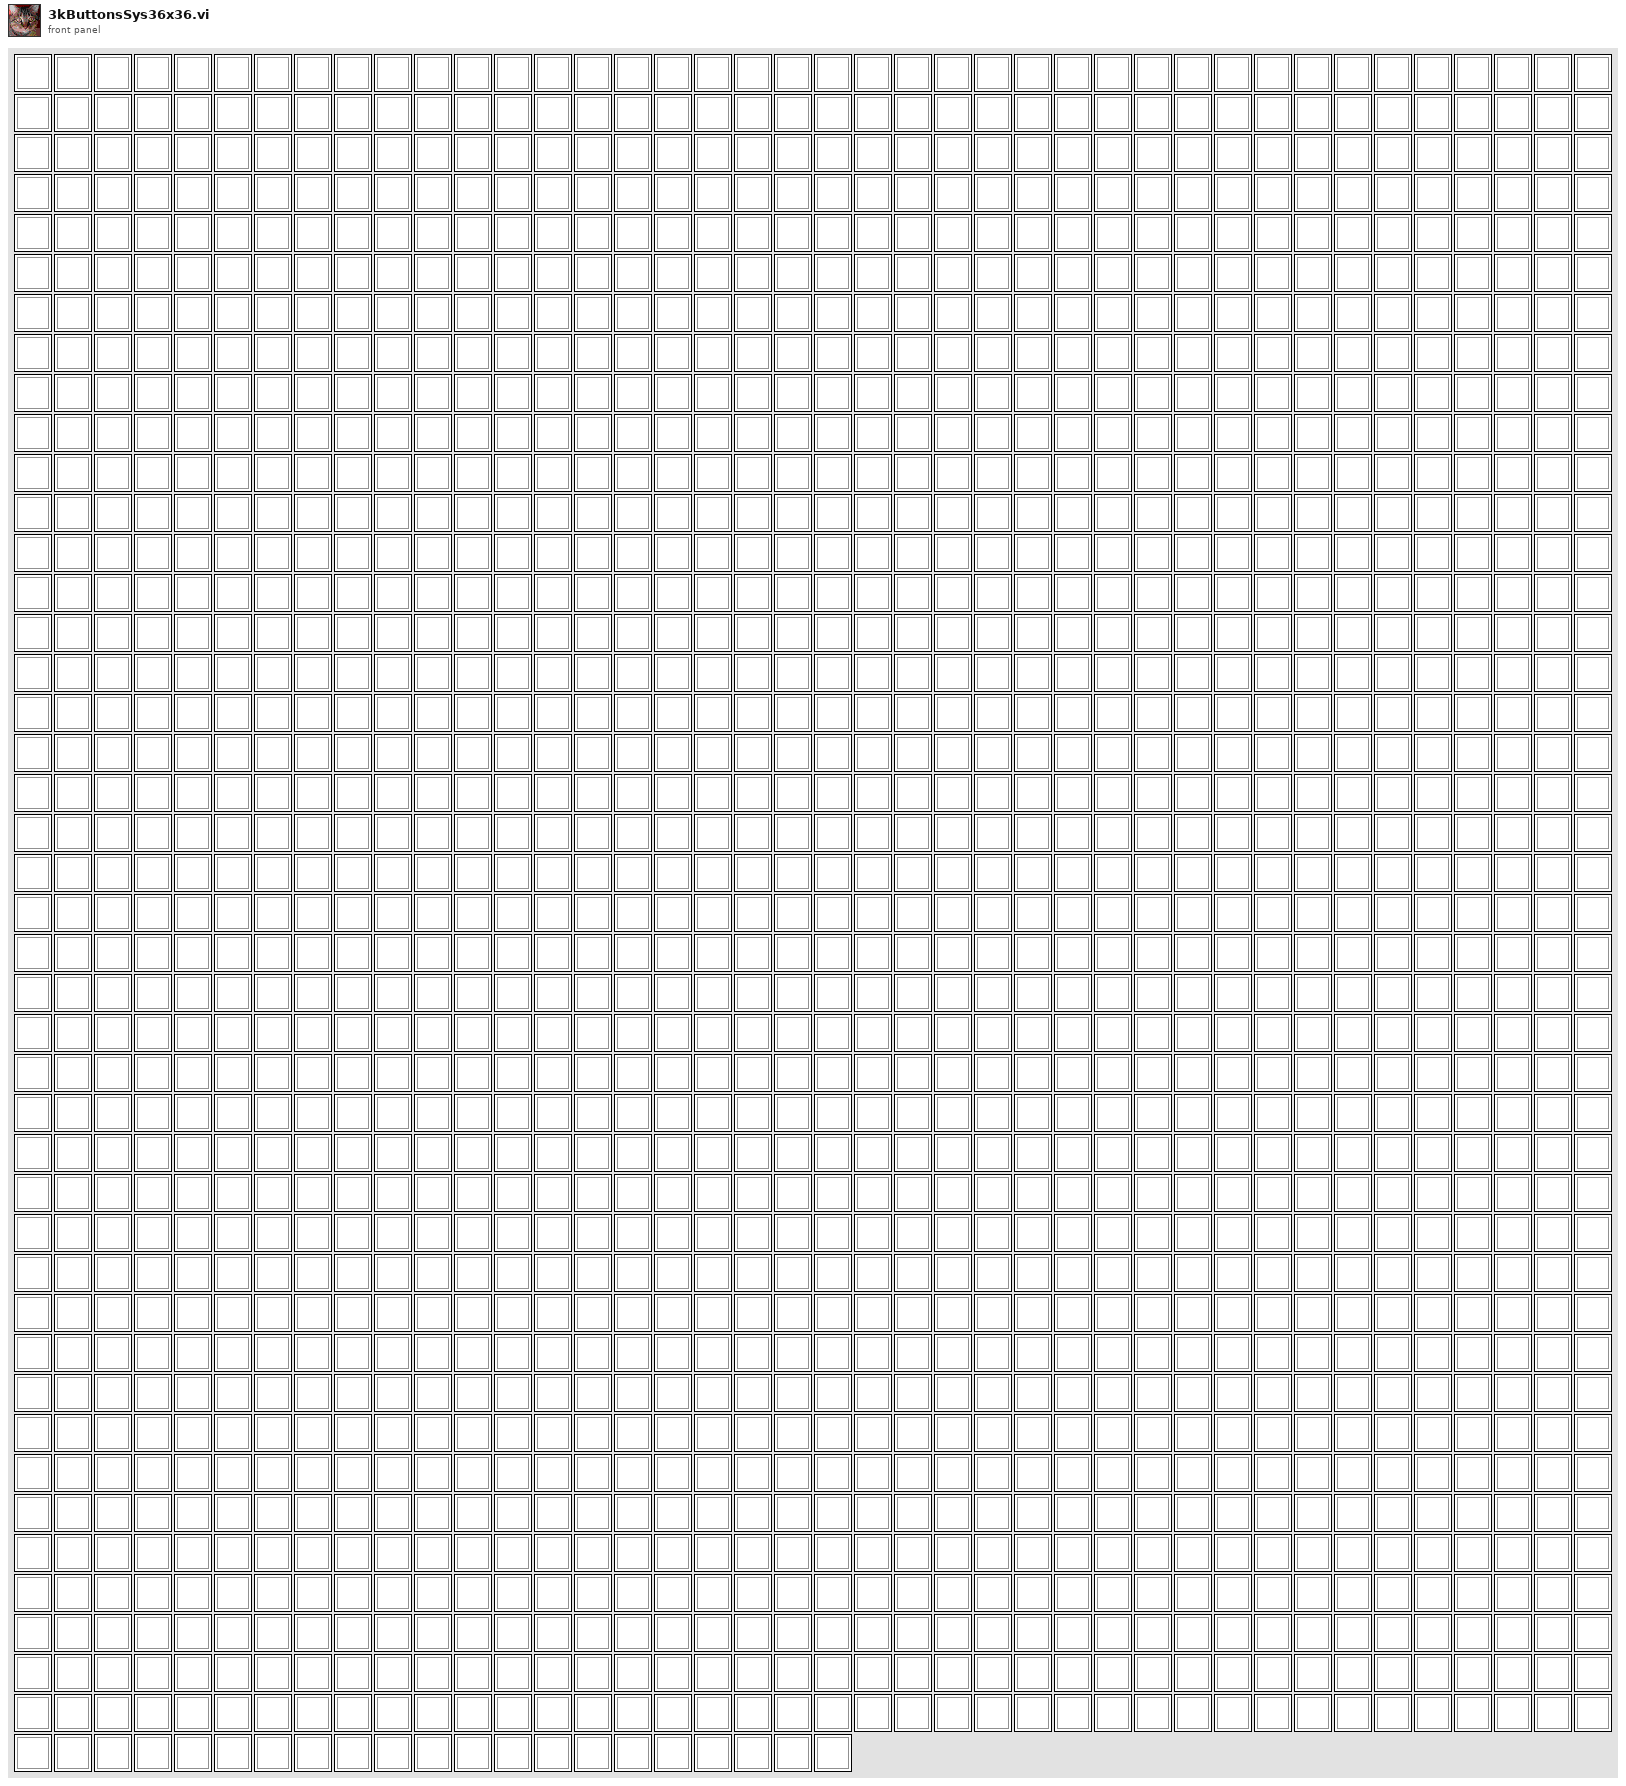
[diagram p1: front panel]
diagram:
